vi "HFRR ADV v040.vi"() -> ()   [LabVIEW 2025] (continued)
                }
                n3121 = for {
                  N: 2 -> [_]
                  tunnel: [w3930] -> w3892
                  tunnel: [w3929] -> w3891
                  tunnel: w3886 -> [w3928]
                  tunnel: w3885 -> [w3927]
                  n3122 = call-dynamic "New Report Line.vi"("report in"=w3928, "error in (no error)"=w3927) -> ("report out"=w3930:refnum<class "NI_report.lvclass">, "error out"=w3929:errorcluster)  [unwired: 12 in]
                }
                n3123 = for {
                  N: 25 -> [_]
                  tunnel: w3892 -> [w3926]
                  tunnel: w3891 -> [w3924]
                  tunnel: [w3925] -> w3895
                  tunnel: [w3923] -> w3894
                  n3124 = call-dynamic "Set Report Tab Width.vi"("report in"=w3926, "error in (no error)"=w3924) -> ("report out"=w3925:refnum<class "NI_report.lvclass">, "error out"=w3923:errorcluster)  [unwired: 12 in]
                }
                n3125 = control-ref of="Tab Control 9"() -> (w3890:refnum<vi>)
                n3126 = call-dynamic "Append Control Image to Report.vi"("report in"=w3895, "alignment (default)"=HTML_Report_Image_Alignment."ABSMIDDLE", "ctrl reference"=w3890, "error in (no error)"=w3894) -> ("report out"=w3889:refnum<class "NI_report.lvclass">, "error out"=w3888:errorcluster)  [unwired: 8 in, 2 out]
                n3127 = for {
                  N: 3 -> [_]
                  tunnel: [w3922] -> w3873
                  tunnel: [w3921] -> w3872
                  tunnel: w3889 -> [w3920]
                  tunnel: w3888 -> [w3919]
                  n3128 = call-dynamic "New Report Line.vi"("report in"=w3920, "error in (no error)"=w3919) -> ("report out"=w3922:refnum<class "NI_report.lvclass">, "error out"=w3921:errorcluster)  [unwired: 12 in]
                }
                n3129 = for {
                  N: 100 -> [_]
                  tunnel: w3873 -> [w3918]
                  tunnel: w3872 -> [w3916]
                  tunnel: [w3917] -> w3869
                  tunnel: [w3915] -> w3867
                  n3130 = call-dynamic "Set Report Tab Width.vi"("report in"=w3918, "error in (no error)"=w3916) -> ("report out"=w3917:refnum<class "NI_report.lvclass">, "error out"=w3915:errorcluster)  [unwired: 12 in]
                }
                n3131 = String To Path(string="C:\\LAB-IQ\\im\\Temp_resized.jpg") -> (path=w3859:path)
                n3132 = call-poly <vilib>:"Append Image to Report.vi"("report in"=w3869, "path or URL of image"=w3859, "error in (no error)"=w3867) -> ("report out"=w3868:refnum<class "NI_report.lvclass">, "error out"=w3866:errorcluster)  [unwired: 9 in, 2 out]
                n3133 = call-poly <vilib>:"Open HTML Report in Browser.vi"("report in"=w3868, "error in (no error)"=w3866) -> ("report out"=w3903:refnum<class "NI_report.lvclass">, "error out"=w3902:errorcluster)  [unwired: 11 in, 1 out]
                n3134 = call-dynamic "Dispose Report.vi"("report in"=w3903, "error in (no error)"=w3902) -> ()  [unwired: 13 in, 1 out]
              }
              frame #2 {
              }
              frame #3 {
                n3135 = disable-structure shown="Disabled" {
                  frame Disabled {
                    n3136 = local read "String 10"() -> (w3943:string)
                    n3137 = Concatenate Strings("C:\\LAB-IQ-NXT\\Data\\" ("string"), w3943, ".jpg" ("string")) -> (w3941:string)
                    n3138 = String To Path(string=w3941) -> (path=w3940:path)
                    n3139 = Delete(path (use dialog)=w3940) -> ()  [unwired: 4 in, 3 out]
                  }
                  frame Enabled {
                  }
                }
                n3140 = local write "Print 2"(FALSE ("Print")) -> ()
              }
            }
          }
        }
      }
    }
    n3141 = Wait (ms)(milliseconds to wait=u32 50) -> ()  [unwired: 1 out]
    n3142 = Wait (ms)(milliseconds to wait=u32 50) -> ()  [unwired: 1 out]
    n3143 = local read "Quit"() -> (w2285:bool)
  }
  n3144 = VISA Close(VISA resource name=w43, error in (no error)=w42) -> ()  [unwired: 1 out]
  n3145 = while {
    stop <- w4094 stop-if-true
    n3146 = local read "Auto Start Test"() -> (w4092:bool)
    n3147 = local read "RUN"() -> (w4091:bool)
    n3148 = Wait (ms)(milliseconds to wait=u32 1000) -> ()  [unwired: 1 out]
    n3149 = Or(x=w4091, y=w4092) -> (x .or. y?=w4090:bool)
    n3150 = case shown="True" w4090 {
      frame False {
      }
      frame True {
        n3151 = local read "LVDT STROKE Actual"() -> (w4095:dbl)
        n3152 = In Range and Coerce(upper limit=1.2, x=w4095, lower limit=0.6) -> (In Range?=w4098:bool)  [unwired: 1 out]
        n3153 = call-poly <vilib>:"Random Number (Range).vi"("lower bound (0)"=0.998 ("upper bound (100)"), "upper bound (100)"=1.003) -> ("number"=w4096:dbl)  [unwired: 9 in]
        n3154 = case shown="True" w4098 {
          tunnel: [w4103 w4104] -> w4097
          tunnel: w4096 -> [_ w4104]
          tunnel: w4095 -> [w4103 _]
          frame False {
          }
          frame True {
          }
        }
        "LVDT STROKE DISPLAY" <- w4097
      }
    }
    n3155 = local read "Quit"() -> (w4094:bool)
  }
  n3156 = while {
    tunnel: [w4121] -> w51
    shift-right: [w4114] -> _
    shift-left: 0.0 -> [w4117]
    shift-right: [w4113] -> _
    shift-left: 0.0 -> [w4116]
    shift-right: [w4112] -> _
    shift-left: 100.0 ("vc_cmd") -> [w4115]
    stop <- w4121 stop-if-true
    # "PID LOGIC"
    n3157 = local read "run test Calibration"() -> (w4109:bool)
    n3158 = local read "RUN"() -> (w4119:bool)
    n3159 = local read "Auto Start Temp"() -> (w4110:bool)
    n3160 = local read "Auto Start Test"() -> (w4118:bool)
    n3161 = local read "START TEMP"() -> (w4108:bool)
    n3162 = And(x=w4110, y=w4118) -> (x .and. y?=w4111:bool)
    n3163 = Or(x=w4119, y=w4111) -> (x .or. y?=w4120:bool)
    n3164 = And(x=w4120, y=w4108) -> (x .and. y?=w4107:bool)
    n3165 = And(x=w4109, y=w4108) -> (x .and. y?=w4106:bool)
    n3166 = Or(x=w4106, y=w4107) -> (x .or. y?=w4105:bool)
    n3167 = Wait (ms)(milliseconds to wait="milliseconds to wait") -> ()  [unwired: 1 out]
    n3168 = case shown="True" w4105 {
      tunnel: [400.0 ("out_vc_cmd") w4140] -> w4112
      tunnel: [w4124 w4142] -> w4113
      tunnel: [w4124 w4141] -> w4114
      tunnel: w4117 -> [_ w4131]
      tunnel: w4116 -> [_ w4130]
      tunnel: w4115 -> [_ w4129]
      tunnel: w4109 -> [_ w4125]
      frame False {
        w4124 = 0.0 ("error_out")
      }
      frame True {
        n3169 = case shown="True" w4125 {
          tunnel: [w4149 1.0] -> w4127
          frame False {
            n3170 = local read "Set Strk"() -> (w4148:dbl)
            n3171 = Add(x=w4148, y="Add up Stroke") -> (x+y=w4149:dbl)
          }
          frame True {
          }
        }
        n3172 = local read "LVDT STROKE"() -> (w4126:dbl)
        n3173 = formula code="// Zero-Hardcode Explicit Positional-Form PID Engine\n// Inputs: target_stroke, measured_stroke, dt, prev_error, integral_accumulator_in, prev_vc_cmd\n//         kp, ki, kd, max_step_change, max_amplitude, min_amplitude, startup_cmd\n// Outputs: vc_cmd, error_out, out_error, integral_accumulator_out, out_vc_cmd\n\n// 1. Calculate Tracking Error\nfloat current_error = target_stroke - measured_stroke;\nerror_out = current_error;\n\n// 2. Compute Proportional Term\nfloat p_term = kp * current_error;\n\n// 3. Compute Derivative Term\nfloat d_term = 0.0;\nif (dt > 0.0) {\n    d_term = kd * ((current_error - prev_error) / dt);\n}\n\n// 4. Update and Accumulate Integral Term\nfloat current_integral = integral_accumulator_in + (current_error * dt);\nfloat i_term = ki * current_integral;\n\n// 5. Calculate Ideal Target Command (Anchored by startup baseline)\nfloat ideal_command = startup_cmd + p_term + i_term + d_term;\n\n// 6. Apply Loop Rate Limiting FIRST \n// (Forces the command to climb gradually from prev_vc_cmd instead of jumping straight to max)\nfloat raw_adjustment = ideal_command - prev_vc_cmd;\n\nif (raw_adjustment > max_step_change) {\n    raw_adjustment = max_step_change;\n} else if (raw_adjustment < -max_step_change) {\n    raw_adjustment = -max_step_change;\n}\n\nfloat next_vc_cmd = prev_vc_cmd + raw_adjustment;\n\n// 7. Anti-Windup Protection & Final Output Safety Safeguard Clamping\n// (Back-calculating based on what we are ACTUALLY outputting)\nif (next_vc_cmd > max_amplitude) {\n    float excess = next_vc_cmd - max_amplitude;\n    if (ki > 0.0) {\n        current_integral -= excess / ki;\n    }\n    next_vc_cmd = max_amplitude;\n} else if (next_vc_cmd < min_amplitude) {\n    float excess = next_vc_cmd - min_amplitude;\n    if (ki > 0.0) {\n        current_integral -= excess / ki;\n    }\n    next_vc_cmd = min_amplitude;\n}\n\n// 8. Map to Shift Registers for memory persistence\nvc_cmd = next_vc_cmd;\nout_error = current_error;                   \nintegral_accumulator_out = current_integral;  \nout_vc_cmd = next_vc_cmd;"("target_stroke"=w4127, "measured_stroke"=w4126, "dt"="dt", "integral_accumulator_in"=w4130, "prev_error"=w4131, "prev_vc_cmd"=w4129, "kp"="kp", "ki"="ki", "kd"="kd", "max_step_change"="max_step_change", "max_amplitude"="max_amplitude", "min_amplitude"="min_amplitude", "startup_cmd"="startup_cmd") -> ("vc_cmd"=w4146:dbl, "out_error"=w4141:dbl, "integral_accumulator_out"=w4142:dbl, "out_vc_cmd"=w4140:dbl)  [unwired: 1 out]
        "output Vpp" <- w4146
        n3174 = Number To Fractional String(number=w4146, precision (6)=i16 1) -> (F-format string=w4144:string)  [unwired: 2 in]
        n3175 = Concatenate Strings("DAC;" ("string"), w4144) -> (w4128:string)
        n3176 = local write "Due Write"(w4128) -> ()
        "prev_error" <- w4131
        "integral_accumulator_in" <- w4130
        "prev_vc_cmd" <- w4129
      }
    }
    n3177 = local read "Quit"() -> (w4121:bool)
  }
  n3178 = Or(x=w47, y=w46) -> (x .or. y?=w48:bool)
  n3179 = Or(x=w44, y=w48) -> (x .or. y?=w53:bool)
  n3180 = control-ref of="new picture"() -> ()  [unwired: 1 out]
  n3181 = Or(x=w56, y=w53) -> (x .or. y?=w50:bool)
  n3182 = Or(x=w50, y=w51) -> (x .or. y?=w45:bool)
  n3183 = while {
    tunnel: [w4151] -> w55
    i -> [w4158]
    stop <- w4151 stop-if-true
    n3184 = local read "Quit"() -> (w4151:bool)
    n3185 = Equal To 0?(x=w4158) -> (x = 0?=w4156:bool)
    n3186 = call "Elapsed Time3"("Time Target (s)"=45.0, "Auto Reset"=TRUE) -> ("Time has Elapsed"=w4155:bool)  [unwired: 10 in, 7 out]
    n3187 = Wait (ms)(milliseconds to wait=u32 50) -> ()  [unwired: 1 out]
    n3188 = Or(x=w4155, y=w4156) -> (x .or. y?=w4157:bool)
    n3189 = case shown="True" w4157 {
      frame False {
      }
      frame True {
        n3190 = call <vilib>:"System Exec.vi"("run minimized? (F)"=TRUE, "error in (no error)"="error in (no error)", "command line"="powercfg.exe -change -monitor-timeout-ac 0") -> ("error out"=w4169:errorcluster)  [unwired: 5 in, 3 out]
        n3191 = call <vilib>:"System Exec.vi"("run minimized? (F)"=TRUE, "error in (no error)"=w4169, "command line"="powercfg.exe -change -disk-timeout-ac 0") -> ("error out"=w4168:errorcluster)  [unwired: 5 in, 3 out]
        n3192 = call <vilib>:"System Exec.vi"("run minimized? (F)"=TRUE, "error in (no error)"=w4168, "command line"="powercfg.exe -change -standby-timeout-ac 0") -> ("error out"=w4167:errorcluster)  [unwired: 5 in, 3 out]
        n3193 = call <vilib>:"System Exec.vi"("run minimized? (F)"=TRUE, "error in (no error)"=w4167, "command line"="powercfg.exe -change -hibernate-timeout-ac 0") -> ("error out"=w4166:errorcluster)  [unwired: 5 in, 3 out]
        n3194 = call <vilib>:"Simple Error Handler.vi"("error in (no error)"=w4166) -> ("error out"=w4172:errorcluster)  [unwired: 4 in, 4 out]
        n3195 = call <vilib>:"Clear Errors.vi"("error in (no error)"=w4172) -> ("error out"=→"error out":errorcluster)  [unwired: 5 in, 1 out]
      }
    }
  }
  n3196 = Compound Arithmetic op=OR(w58, w45, w55) -> (w57:bool)
  n3197 = flat-sequence {
    tunnel: w57 -> [_]
    tunnel: [w4174] -> w27
    tunnel: w27 -> [_]
    frame #0 {
      n3198 = call "CLOSE CONNECTION.vi"() -> ("error out"=w4174:errorcluster)  [unwired: 11 in]
    }
    frame #1 {
      n3199 = Quit LabVIEW(quit? (T)=TRUE) -> ()
      n3200 = local write "Quit"(FALSE ("EXIT")) -> ()
    }
  }
  n3201 = property on="Heater Button" class="Bool (strict)"("Visible"=TRUE) -> ()  [unwired: 2 in, 2 out]
  n3202 = while {
    tunnel: [w4181] -> _
    i -> [w4181]
    stop <- w4177 stop-if-true
    # "Langauage selection"
    n3203 = Equal?(x="Lan flag", y=22.0) -> ()  [unwired: 1 out]
    n3204 = disable-structure shown="Disabled" {
      frame Disabled {
        n3205 = stacked-sequence {
          frame #0 {
            n3206 = case shown="\"Russian\"" "Language Selection" {
              tunnel: [0 1] -> w4183
              frame "English", Default {
              }
              frame "Russian" {
              }
            }
            n3207 = for {
              N: 130 -> [_]
              tunnel: "Table" -> [w4192]
              tunnel: w4183 -> [w4191]
              i -> [w4190]
              n3208 = Index Array(array=w4192, index (row)=w4190, index (col)=w4191) -> (element=w4189:string)
              n3209 = case shown="1" w4190 {
                tunnel: w4189 -> [w4193 w4194 _ w4195 w4196 w4197 w4198 w4199 w4200 w4201 w4202 w4203 w4204 w4205 w4206 w4207 w4208 w4209 w4210 w4211 w4212 w4213 w4214 w4215 w4216 w4217 w4218 w4219 w4220 _ _ w4221 w4222 w4223 w4224 w4225 w4226 w4235 w4242 w4249 w4256 w4260 w4263 w4266 w4268 w4270 w4271 w4272 w4273 w4274 w4275 w4276 w4277 w4278 w4279 w4280 w4281 w4282 w4283 w4284 w4285 w4286 w4287 w4288 w4289 w4290 w4291 w4292 w4293 w4294 w4295 w4296 w4297 w4298 w4299 w4300 w4301 w4302 w4303 w4304 w4305 w4306 w4307 w4308 w4309 w4310 w4311 w4312 w4313 w4314 w4315 w4316 w4317 w4318 w4319 w4320 w4321 w4322 w4323 w4324 w4325 w4326 w4327 w4328 w4329 _ w4330 w4331 w4332 w4333 w4334 w4335 w4336 w4337 w4338 w4339 w4340 w4341 w4342 _ w4343 w4344 w4345 w4346 w4347 w4348 _]
                frame 0 {
                  n3210 = local write "S"(w4193) -> ()
                }
                frame 1 {
                  n3211 = local write "S 2"(w4194) -> ()
                }
                frame 2 {
                }
                frame 3 {
                  n3212 = local write "S 4"(w4195) -> ()
                }
                frame 4 {
                  n3213 = property on="FILE" class="Str"("Caption.Text"=w4196) -> ()  [unwired: 2 in, 2 out]
                }
                frame 5 {
                  n3214 = property on="Fuel Discription :" class="Str"("Caption.Text"=w4197) -> ()  [unwired: 2 in, 2 out]
                }
                frame 6 {
                  n3215 = property on="Remarks :" class="Str"("Caption.Text"=w4198) -> ()  [unwired: 2 in, 2 out]
                }
                frame 7 {
                  n3216 = property on="Save & Continue" class="Bool (strict)"("Boolean Text.Text"=w4199) -> ()  [unwired: 2 in, 2 out]
                }
                frame 8 {
                }
                frame 9 {
                  n3217 = property on="Set Hz" class="DigNum (strict)"("Caption.Text"=w4201) -> ()  [unwired: 2 in, 2 out]
                }
                frame 10 {
                }
                frame 11 {
                  n3218 = property on="NORMAL LOAD" class="DigNum (strict)"("Caption.Text"=w4203) -> ()  [unwired: 2 in, 2 out]
                }
                frame 12 {
                }
                frame 13 {
                  n3219 = property on="Set Temp" class="DigNum (strict)"("Caption.Text"=w4205) -> ()  [unwired: 2 in, 2 out]
                }
                frame 14 {
                  n3220 = local write "S 15"(w4206) -> ()
                }
                frame 15 {
                  n3221 = property on="Set Rh" class="DigNum (strict)"("Caption.Text"=w4207) -> ()  [unwired: 2 in, 2 out]
                }
                frame 16 {
                }
                frame 17 {
                  n3222 = local write "S 18"(w4209) -> ()
                }
                frame 18 {
                  "String 17" <- w4210
                }
                frame 19 {
                  n3223 = property on="test time" class="DigNum (strict)"("Caption.Text"=w4211) -> ()  [unwired: 2 in, 2 out]
                }
                frame 20 {
                  "String 18" <- w4212
                  "String 22" <- w4212
                }
                frame 21 {
                  n3224 = property on="Elapsed time" class="DigNum (strict)"("Caption.Text"=w4213) -> ()  [unwired: 2 in, 2 out]
                }
                frame 22 {
                  n3225 = property on="Samplingtime 2" class="DigNum (strict)"("Caption.Text"=w4214) -> ()  [unwired: 2 in, 2 out]
                }
                frame 23 {
                  "String 21" <- w4215
                }
                frame 24 {
                  n3226 = property on="Countdown" class="DigNum (strict)"("Caption.Text"=w4216) -> ()  [unwired: 2 in, 2 out]
                }
                frame 25 {
                  n3227 = property on="Countdown 2" class="DigNum (strict)"("Caption.Text"=w4217) -> ()  [unwired: 2 in, 2 out]
                }
                frame 26 {
                  n3228 = property on="Engage" class="Bool (strict)"("Boolean Text.Text"=w4218) -> ()  [unwired: 2 in, 2 out]
                }
                frame 27 {
                  n3229 = property on="Boolean  4" class="Bool (strict)"("Boolean Text.Text"=w4219) -> ()  [unwired: 2 in, 2 out]
                }
                frame 28 {
                  n3230 = property on="Test \nStatus" class="Bool (strict)"("Boolean Text.Text"=w4220) -> ()  [unwired: 2 in, 2 out]
                }
                frame 29 {
                }
                frame 30 {
                }
                frame 31 {
                }
                frame 32 {
                  n3231 = property on="RSTCOF" class="Bool"("Boolean Text.Text"=w4222) -> ()  [unwired: 2 in, 2 out]
                  n3232 = property on="RST FF" class="Bool"("Boolean Text.Text"=w4222) -> ()  [unwired: 2 in, 2 out]
                  n3233 = property on="RST TEMP" class="Bool"("Boolean Text.Text"=w4222) -> ()  [unwired: 2 in, 2 out]
                  n3234 = property on="RSTV1 3" class="Bool"("Boolean Text.Text"=w4222) -> ()  [unwired: 2 in, 2 out]
                  n3235 = property on="rstv2" class="Bool"("Boolean Text.Text"=w4222) -> ()  [unwired: 2 in, 2 out]
                  n3236 = property on="RSTV1 2" class="Bool"("Boolean Text.Text"=w4222) -> ()  [unwired: 2 in, 2 out]
                  n3237 = property on="RST CP" class="Bool"("Boolean Text.Text"=w4222) -> ()  [unwired: 2 in, 2 out]
                }
                frame 33 {
                  "S 61" <- w4223
                }
                frame 34 {
                  "String 23" <- w4224
                }
                frame 35 {
                  n3238 = property on="Rh Before" class="DigNum (strict)"("Caption.Text"=w4225) -> ()  [unwired: 2 in, 2 out]
                }
                frame 36 {
                  n3239 = Match Pattern(string=w4226, regular expression=",") -> (before substring=→"bs":string, after substring=→"as":string)  [unwired: 1 in, 2 out]
                  n3240 = property on="Rh After" class="DigNum (strict)"("Caption.Text"=w4226) -> ()  [unwired: 2 in, 2 out]
                }
                frame 37 {
                  n3241 = Match Pattern(string=w4235, regular expression=",") -> (before substring=w4234:string, after substring=w4233:string)  [unwired: 1 in, 2 out]
                  "bs" <- w4234
                  "as" <- w4233
                  n3242 = Concatenate Strings(w4234, w4233) -> (w4230:string)
                  n3243 = property on="Humidity before test 2" class="DigNum (strict)"("Caption.Text"=w4230) -> ()  [unwired: 2 in, 2 out]
                  n3244 = Concatenate Strings(w4230, "=" ("string")) -> (w4231:string)
                  n3245 = local write "S 38"(w4231) -> ()
                }
                frame 38 {
                  n3246 = Match Pattern(string=w4242, regular expression=",") -> (before substring=w4241:string, after substring=w4240:string)  [unwired: 1 in, 2 out]
                  "bs" <- w4241
                  "as" <- w4240
                  n3247 = Concatenate Strings(w4241, w4240) -> (w4237:string)
                  n3248 = property on="Humidity after test 2" class="DigNum (strict)"("Caption.Text"=w4237) -> ()  [unwired: 2 in, 2 out]
                  n3249 = Concatenate Strings(w4237, "=" ("string")) -> (w4239:string)
                  n3250 = local write "S 39"(w4239) -> ()
                }
                frame 39 {
                  n3251 = Match Pattern(string=w4249, regular expression=",") -> (before substring=w4248:string, after substring=w4247:string)  [unwired: 1 in, 2 out]
                  "bs" <- w4248
                  "as" <- w4247
                  n3252 = Concatenate Strings(w4248, w4247) -> (w4244:string)
                  n3253 = property on="Temperature before test 2" class="DigNum (strict)"("Caption.Text"=w4244) -> ()  [unwired: 2 in, 2 out]
                  n3254 = Concatenate Strings(w4244, "=" ("string")) -> (→"String 34":string)
                }
                frame 40 {
                  n3255 = Match Pattern(string=w4256, regular expression=",") -> (before substring=w4255:string, after substring=w4254:string)  [unwired: 1 in, 2 out]
                  "bs" <- w4255
                  "as" <- w4254
                  n3256 = Concatenate Strings(w4255, w4254) -> (w4251:string)
                  n3257 = property on="Temperature after test 2" class="DigNum (strict)"("Caption.Text"=w4251) -> ()  [unwired: 2 in, 2 out]
                  n3258 = Concatenate Strings(w4251, "=" ("string")) -> (→"String 35":string)
                  n3259 = property on="Temperature after test" class="DigNum (strict)"("Caption.Text"=w4251) -> ()  [unwired: 2 in, 2 out]
                }
                frame 41 {
                  n3260 = property on="AVP 2" class="DigNum (strict)"("Caption.Text"=w4260) -> ()  [unwired: 2 in, 2 out]
                  n3261 = Concatenate Strings(w4260, "=" ("string")) -> (→"String 36":string)
                }
                frame 42 {
                  n3262 = property on="MWSD 2" class="DigNum (strict)"("Caption.Text"=w4263) -> ()  [unwired: 2 in, 2 out]
                  n3263 = Concatenate Strings(w4263, "=" ("string")) -> (→"String 37":string)
                }
                frame 43 {
                  n3264 = property on="HCF 2" class="DigNum (strict)"("Caption.Text"=w4266) -> ()  [unwired: 2 in, 2 out]
                  n3265 = Concatenate Strings(w4266, "=" ("string")) -> (→"String 38":string)
                }
                frame 44 {
                  n3266 = Concatenate Strings(w4268, "=" ("string")) -> (→"String 39":string)
                  n3267 = property on="WS1.4 2" class="DigNum (strict)"("Caption.Text"=w4268) -> ()  [unwired: 2 in, 2 out]
                }
                frame 45 {
                }
                frame 46 {
                  n3268 = local write "S 47"(w4271) -> ()
                }
                frame 47 {
                  n3269 = local write "S 48"(w4272) -> ()
                }
                frame 48 {
                  n3270 = local write "S 49"(w4273) -> ()
                }
                frame 49 {
                  n3271 = local write "S 50"(w4274) -> ()
                }
                frame 50 {
                  n3272 = local write "S 51"(w4275) -> ()
                }
                frame 51 {
                  n3273 = local write "S 52"(w4276) -> ()
                }
                frame 52 {
                  n3274 = local write "S 53"(w4277) -> ()
                }
                frame 53 {
                  n3275 = local write "S 54"(w4278) -> ()
                }
                frame 54 {
                  n3276 = local write "S 55"(w4279) -> ()
                }
                frame 55 {
                  n3277 = local write "S 56"(w4280) -> ()
                }
                frame 56 {
                  n3278 = local write "S 57"(w4281) -> ()
                }
                frame 57 {
                  n3279 = local write "S 58"(w4282) -> ()
                }
                frame 58 {
                  n3280 = local write "S 59"(w4283) -> ()
                }
                frame 59 {
                  n3281 = local write "S 60"(w4284) -> ()
                }
                frame 60 {
                  n3282 = local write "S 62"(w4285) -> ()
                }
                frame 61 {
                  n3283 = local write "S 63"(w4286) -> ()
                }
                frame 62 {
                  n3284 = local write "S 64"(w4287) -> ()
                }
                frame 63 {
                  n3285 = local write "S 65"(w4288) -> ()
                }
                frame 64 {
                  n3286 = local write "S 66"(w4289) -> ()
                }
                frame 65 {
                  n3287 = local write "S 67"(w4290) -> ()
                }
                frame 66 {
                  n3288 = local write "S 68"(w4291) -> ()
                }
                frame 67 {
                  n3289 = local write "S 69"(w4292) -> ()
                }
                frame 68 {
                  n3290 = local write "S 70"(w4293) -> ()
                }
                frame 69 {
                  n3291 = local write "S 71"(w4294) -> ()
                }
                frame 70 {
                  n3292 = local write "S 72"(w4295) -> ()
                }
                frame 71 {
                  n3293 = local write "S 73"(w4296) -> ()
                }
                frame 72 {
                  n3294 = local write "S 74"(w4297) -> ()
                }
                frame 73 {
                  n3295 = local write "S 75"(w4298) -> ()
                }
                frame 74 {
                  n3296 = local write "S 76"(w4299) -> ()
                }
                frame 75 {
                  n3297 = local write "S 77"(w4300) -> ()
                }
                frame 76 {
                  n3298 = local write "S 78"(w4301) -> ()
                }
                frame 77 {
                  n3299 = local write "S 79"(w4302) -> ()
                }
                frame 79 {
                  n3300 = property on="Sample Temperature ( °C )" class="XYGraph (strict)"("Y Scale.Name Label.Text"=w4303) -> ()  [unwired: 2 in, 2 out]
                }
                frame 80 {
                  n3301 = local write "S 81"(w4304) -> ()
                  n3302 = property on="Humidity ( %RH )" class="XYGraph (strict)"("Y Scale.Name Label.Text"=w4304) -> ()  [unwired: 2 in, 2 out]
                }
                frame 78 {
                  n3303 = property on="Air Temperature  ( °C )" class="XYGraph (strict)"("X Scale.Name Label.Text"=w4305) -> ()  [unwired: 2 in, 2 out]
                  n3304 = property on="Humidity ( %RH )" class="XYGraph (strict)"("X Scale.Name Label.Text"=w4305) -> ()  [unwired: 2 in, 2 out]
                  n3305 = property on="Sample Temperature ( °C )" class="XYGraph (strict)"("X Scale.Name Label.Text"=w4305) -> ()  [unwired: 2 in, 2 out]
                  n3306 = property on="Coefficient Of Friction" class="XYGraph (strict)"("X Scale.Name Label.Text"=w4305) -> ()  [unwired: 2 in, 2 out]
                }
                frame 81 {
                  n3307 = property on="Air Temperature  ( °C )" class="XYGraph (strict)"("Y Scale.Name Label.Text"=w4306) -> ()  [unwired: 2 in, 2 out]
                }
                frame 82 {
                  n3308 = local write "S 84"(w4307) -> ()
                }
                frame 83 {
                  n3309 = local write "S 85"(w4308) -> ()
                }
                frame 84 {
                  n3310 = local write "S 86"(w4309) -> ()
                }
                frame 85 {
                  n3311 = local write "S 87"(w4310) -> ()
                }
                frame 86 {
                  n3312 = local write "S 88"(w4311) -> ()
                }
                frame 87 {
                }
                frame 88 {
                  n3313 = local write "S 90"(w4313) -> ()
                }
                frame 89 {
                  n3314 = local write "S 91"(w4314) -> ()
                }
                frame 90 {
                  n3315 = local write "S 92"(w4315) -> ()
                }
                frame 91 {
                  n3316 = local write "S 93"(w4316) -> ()
                }
                frame 92 {
                  n3317 = local write "S 94"(w4317) -> ()
                }
                frame 93 {
                  n3318 = local write "S 95"(w4318) -> ()
                }
                frame 94 {
                  n3319 = local write "S 96"(w4319) -> ()
                }
                frame 95 {
                  n3320 = local write "S 97"(w4320) -> ()
                }
                frame 96 {
                  n3321 = local write "S 98"(w4321) -> ()
                }
                frame 97 {
                  n3322 = local write "S 99"(w4322) -> ()
                }
                frame 98 {
                  n3323 = local write "S 100"(w4323) -> ()
                }
                frame 99 {
                  n3324 = local write "S 101"(w4324) -> ()
                }
                frame 100 {
                  n3325 = local write "S 102"(w4325) -> ()
                }
                frame 101 {
                  n3326 = local write "S 103"(w4326) -> ()
                }
                frame 102 {
                  n3327 = local write "S 104"(w4327) -> ()
                }
                frame 103 {
                  n3328 = local write "S 105"(w4328) -> ()
                }
                frame 104 {
                  n3329 = local write "S 106"(w4329) -> ()
                }
                frame 105 {
                }
                frame 106 {
                  n3330 = property on="OK Button 17" class="Bool (strict)"("Boolean Text.Text"=w4330) -> ()  [unwired: 2 in, 2 out]
                }
                frame 107 {
                  n3331 = property on="OK Button 16" class="Bool (strict)"("Boolean Text.Text"=w4331) -> ()  [unwired: 2 in, 2 out]
                }
                frame 108 {
                  n3332 = property on="TITTLE" class="Str"("Caption.Text"=w4332) -> ()  [unwired: 2 in, 2 out]
                }
                frame 109 {
                  "String 30" <- w4333
                }
                frame 110 {
                  n3333 = property on="Test Date" class="Str"("Caption.Text"=w4334) -> ()  [unwired: 2 in, 2 out]
                  "String 31" <- w4334
                }
                frame 111 {
                  n3334 = property on="Sample ID" class="Str"("Caption.Text"=w4335) -> ()  [unwired: 2 in, 2 out]
                  "String 32" <- w4335
                }
                frame 112 {
                  n3335 = property on="Tested by" class="Str"("Caption.Text"=w4336) -> ()  [unwired: 2 in, 2 out]
                  "String 33" <- w4336
                }
                frame 113 {
                  n3336 = property on="System Configured Printers 2" class="Arr (strict)"("Caption.Text"=w4337) -> ()  [unwired: 2 in, 2 out]
                }
                frame 114 {
                  n3337 = property on="Selected Printer" class="Str"("Caption.Text"=w4338) -> ()  [unwired: 2 in, 2 out]
                }
                frame 115 {
                  n3338 = property on="Select Printer 3" class="DigNum (strict)"("Caption.Text"=w4339) -> ()  [unwired: 2 in, 2 out]
                }
                frame 116 {
                  n3339 = property on="Print" class="Bool (strict)"("Boolean Text.Text"=w4340) -> ()  [unwired: 2 in, 2 out]
                }
                frame 117 {
                  "String 41" <- w4341
                }
                frame 118 {
                  n3340 = property on="tested by" class="Str"("Caption.Text"=w4342) -> ()  [unwired: 2 in, 2 out]
                }
                frame 119 {
                }
                frame 120 {
                  n3341 = property on="Export" class="Bool (strict)"("Boolean Text.Text"=w4343) -> ()  [unwired: 2 in, 2 out]
                }
                frame 121 {
                }
                frame 122 {
                }
                frame 123 {
                  n3342 = property on="Select File Type" class="Enum (strict)"("Caption.Text"=w4346) -> ()  [unwired: 2 in, 2 out]
                }
                frame 124 {
                  n3343 = property on="s.NO" class="Str"("Caption.Text"=w4347) -> ()  [unwired: 2 in, 2 out]
                  "String 45" <- w4347
                }
                frame 125 {
                  n3344 = property on="trip1 8" class="Bool (strict)"("Boolean Text.Text"=w4348) -> ()  [unwired: 2 in, 2 out]
                }
                frame 126, Default {
                }
              }
            }
          }
          frame #1 {
            w4356 = TRUE ("Visible")
            n3345 = local read "S 91"() -> (w4373:string)
            n3346 = local read "S 90"() -> (w4372:string)
            n3347 = local read "S 88"() -> (w4371:string)
            n3348 = property on="File Path" class="Path"("Caption.Text"=w4372) -> ()  [unwired: 2 in, 2 out]
            n3349 = local read "S 71"() -> (w4366:string)
            n3350 = local read "S 86"() -> (w4368:string)
            n3351 = local read "S 85"() -> (w4369:string)
            n3352 = local read "S 87"() -> (w4367:string)
            n3353 = local read "S 84"() -> (w4370:string)
            n3354 = local read "S 103"() -> (w4355:string)
            n3355 = local read "S 104"() -> (w4354:string)
            n3356 = property on="Password" class="Str"("Caption.Text"=w4369) -> ()  [unwired: 2 in, 2 out]
            n3357 = property on="EDIT" class="Bool (strict)"("Boolean Text.Text"=w4366) -> ()  [unwired: 2 in, 2 out]
            n3358 = property on="SAVE" class="Bool (strict)"("Boolean Text.Text"=w4370) -> ()  [unwired: 2 in, 2 out]
            n3359 = Build Array(w4355, w4354) -> (w4353:string[])
            n3360 = property on="Heater Button" class="Bool (strict)"("Strings [4]"=w4353) -> ()  [unwired: 2 in, 2 out]
            n3361 = local read "S 92"() -> (w4365:string)
            n3362 = local read "S 93"() -> (w4364:string)
            n3363 = local read "S 105"() -> (w4351:string)
            n3364 = local read "S 106"() -> (w4350:string)
            n3365 = Build Array(w4365, w4364) -> ()  [unwired: 1 out]
            n3366 = Build Array(w4351, w4350) -> (w4352:string[])
            n3367 = local read "S 95"() -> (w4362:string)
            n3368 = local read "S 94"() -> (w4363:string)
            n3369 = local read "bs"() -> (w4378:string)
            n3370 = local read "as"() -> (w4379:string)
            n3371 = property on="Humidity" class="Bool (strict)"("Strings [4]"=w4352) -> ()  [unwired: 2 in, 2 out]
            n3372 = Concatenate Strings(w4378, "\r", w4379) -> ()  [unwired: 1 out]
            n3373 = property on="Rh After" class="DigNum (strict)"("Caption.Size to Text?"=TRUE ("Caption.Size to Text")) -> ()  [unwired: 2 in, 2 out]
            n3374 = local read "S 48"() -> (w4402:string)
            n3375 = local read "S 50"() -> (w4400:string)
            n3376 = local read "S 51"() -> (w4399:string)
            n3377 = local read "S 49"() -> (w4401:string)
            n3378 = local read "S 52"() -> (w4398:string)
            n3379 = local read "as"() -> (w4383:string)
            n3380 = local read "bs"() -> (w4384:string)
            n3381 = local read "S 56"() -> (w4397:string)
            n3382 = local read "S 57"() -> (w4396:string)
            n3383 = local read "S 58"() -> (w4395:string)
            n3384 = local read "S 59"() -> (w4394:string)
            n3385 = property on="OPEN" class="Bool (strict)"("Boolean Text.Text"=w4398) -> ()  [unwired: 2 in, 2 out]
            n3386 = property on="OPEN 1" class="Bool (strict)"("Boolean Text.Text"=w4402) -> ()  [unwired: 2 in, 2 out]
            n3387 = property on="OPEN 2" class="Bool (strict)"("Boolean Text.Text"=w4401) -> ()  [unwired: 2 in, 2 out]
            n3388 = property on="OPEN 3" class="Bool (strict)"("Boolean Text.Text"=w4400) -> ()  [unwired: 2 in, 2 out]
            n3389 = property on="OPEN 4" class="Bool (strict)"("Boolean Text.Text"=w4399) -> ()  [unwired: 2 in, 2 out]
            n3390 = Concatenate Strings(w4384, "\r", w4383) -> ()  [unwired: 1 out]
            n3391 = local read "S 102"() -> (w4357:string)
            n3392 = property on="КОФ1" class="DigNum (strict)"("Caption.Text"=w4397) -> ()  [unwired: 2 in, 2 out]
            n3393 = local read "S 98"() -> (w4361:string)
            n3394 = local read "S 99"() -> (w4360:string)
            n3395 = local read "S 100"() -> (w4359:string)
            n3396 = local read "S 101"() -> (w4358:string)
            n3397 = property on="КОФ2" class="DigNum (strict)"("Caption.Text"=w4396) -> ()  [unwired: 2 in, 2 out]
            n3398 = property on="КОФ3" class="DigNum (strict)"("Caption.Text"=w4395) -> ()  [unwired: 2 in, 2 out]
            n3399 = property on="КОФ4" class="DigNum (strict)"("Caption.Text"=w4394) -> ()  [unwired: 2 in, 2 out]
            n3400 = local read "bs"() -> (w4382:string)
            n3401 = local read "as"() -> (w4381:string)
            n3402 = local read "S 60"() -> (w4393:string)
            n3403 = local read "S 54"() -> (w4403:string)
            n3404 = Concatenate Strings(w4382, "\r", w4381) -> ()  [unwired: 1 out]
            n3405 = Concatenate Strings(w4403, w4393) -> ()  [unwired: 1 out]
            n3406 = local read "S 77"() -> (→"String 43":string)
            n3407 = local read "S 76"() -> (w4376:string)
            n3408 = local read "S 78"() -> (w4375:string)
            n3409 = local read "S 71"() -> (w4387:string)
            n3410 = local read "S 66"() -> (w4392:string)
            n3411 = local read "S 67"() -> (w4391:string)
            n3412 = local read "S 68"() -> (w4390:string)
            n3413 = local read "S 69"() -> (w4389:string)
            n3414 = local read "S 70"() -> (w4388:string)
            n3415 = property on="AIR TEMP" class="DigNum (strict)"("Caption.Text"=w4375) -> ()  [unwired: 2 in, 2 out]
            n3416 = property on="Set Strk" class="DigNum (strict)"("Caption.Text"=w4376) -> ()  [unwired: 2 in, 2 out]
            n3417 = property on="SPEED OUT:" class="DigNum (strict)"("Caption.Text"=w4390) -> ()  [unwired: 2 in, 2 out]
            n3418 = property on="EDIT" class="Bool (strict)"("Boolean Text.Text"=w4387) -> ()  [unwired: 2 in, 2 out]
            n3419 = local read "S 79"() -> (w4374:string)
          }
          frame #2 {
          }
        }
        n3420 = local write "Lan flag"(10.0 ("Lan flag")) -> ()
      }
      frame Enabled {
      }
    }
    n3421 = Wait (ms)(milliseconds to wait=u32 2000) -> ()  [unwired: 1 out]
    n3422 = local read "Quit"() -> (w4177:bool)
  }
  n3423 = while {
    shift-right: [w4409] -> _
    shift-left: _ -> [w4410]
    shift-right: [w4407] -> _
    shift-left: T18 {"Read Heave and Surge"="", "Bytes at Heave Port"=0.0, "Heave and Surge COM Port:"="COM9", "Com Port 2"="COM7", "Residual Due"="", "Heave COM Status 2"=TRUE, "Heave COM Status"=TRUE, "Port 2"=TRUE, "Sway PPR"=6400.0, "Surge PPR"=6400.0, "Heave PPR"=6400.0, "Sway Pitch"=2.0, "Surge Pitch"=3.0, "Heave Pitch"=4.0, "Sway Pulses/mm"=320.0, "Surge Pulses/mm"=1600.0, "Heave Pulses/mm"=1600.0, "inner loop"=0.0, "Read Heave and Surge 2"="", "String 36"="", "Write S"=FALSE, "WriteCC1"=[""], "Heave COM Loop"=0, "LastCom"="", "EXIT"=FALSE, "Error Heave"={"status"=TRUE, "code"=-1073807343, "source"=""}} -> [w4406]
    shift-right: [w4404] -> _
    shift-left: enum16{"init", "MAIN", "Panel Close"}."init" -> [w4405]
    stop <- w4408 stop-if-true
    # "HUMIDITY LOOP LOGIC"
    n3424 = case shown="\"MAIN\"" w4405 {
      tunnel: w4410 -> [w4424 w4448 w4512 w4514]
      tunnel: [w4419 w4435 w4512 w4514] -> w4409
      tunnel: [_ _ TRUE _] -> w4408
      tunnel: [w4416 w4433 w4510 w4513] -> w4407
      tunnel: w4406 -> [w4421 w4447 w4510 w4513]
      tunnel: [enum16{"init", "MAIN", "Panel Close"}."MAIN" w4442 _ _] -> w4404
      frame "init" {
        n3425 = local read "C3 :"() -> (w4411:refnum<visa-resource-name>)
        n3426 = Bundle By Name(cluster=w4421, "Heave and Surge COM Port:"=w4411) -> (w4420:T18)
        n3427 = call "Instrument fgv uno.vi"("Enum"=T32."INIT", "error in (no error) 2"=w4424, "INPUT"=w4420) -> ("error"=w4422:errorcluster, "output"=w4418:T18)  [unwired: 6 in, 1 out]
        n3428 = case shown="Error" w4422 {
          selector: w4422 -> [w4426 _]
          tunnel: [w4426 w4430] -> w4419
          tunnel: w4418 -> [w4425 w4428]
          tunnel: [w4425 w4427] -> w4417
          frame No Error {
          }
          frame Error {
            n3429 = call "Instrument fgv uno.vi"("Enum"=T32."ERROR INIT", "INPUT"=w4428) -> ("error"=w4431:errorcluster, "output"=w4427:T18)  [unwired: 7 in, 1 out]
            n3430 = call <vilib>:"Clear Errors.vi"("error in (no error)"=w4431) -> ("error out"=w4430:errorcluster)  [unwired: 5 in, 1 out]
          }
        }
        n3431 = local read "LastCom Humidity"() -> (w4414:string)
        n3432 = Unbundle By Name(w4417) -> ("Heave COM Status 2"=→"COM Status":bool, "Error Heave"=→"Error":errorcluster)  [unwired: 1 out]
        n3433 = Bundle By Name(cluster=w4417, "LastCom"=w4414) -> (w4416:T18)
      }
      frame "MAIN" {
        n3434 = Unbundle By Name(w4447) -> ("Com Port 2"=w4437:refnum<visa-resource-name>)
        n3435 = local read "C3 :"() -> (w4438:refnum<visa-resource-name>)
        n3436 = local write "COM Port Humidity :"(w4437) -> ()
        n3437 = Bundle By Name(cluster=w4447, "Heave and Surge COM Port:"=w4438) -> (w4446:T18)
        n3438 = Equal?(x=w4437, y=w4438) -> (x = y?=w4451:bool)
        n3439 = case shown="True" w4451 {
          tunnel: [w4466 w4483] -> w4436
          tunnel: w4448 -> [w4467 w4489]
          tunnel: w4446 -> [w4465 w4487]
          tunnel: [w4464 w4482] -> w4434
          frame False {
            n3440 = call <vilib>:"Clear Errors.vi"("error in (no error)"=w4467) -> ("error out"=w4463:errorcluster)  [unwired: 5 in, 1 out]
            n3441 = call "Instrument fgv uno.vi"("Enum"=T32."ERROR INIT", "error in (no error) 2"=w4463, "INPUT"=w4465) -> ("error"=w4469:errorcluster, "output"=w4464:T18)  [unwired: 6 in, 1 out]
            n3442 = call <vilib>:"Clear Errors.vi"("error in (no error)"=w4469) -> ("error out"=w4466:errorcluster)  [unwired: 5 in, 1 out]
          }
          frame True {
            n3443 = call "Instrument fgv uno.vi"("Enum"=T32."READ", "error in (no error) 2"=w4489, "INPUT"=w4487) -> ("error"=w4488:errorcluster, "output"=w4481:T18)  [unwired: 6 in, 1 out]
            n3444 = Bundle By Name(cluster=w4481, "String 36"="WRITE HUMIDITY") -> (w4480:T18)
            n3445 = case shown="True" "Write Humidity" {
              selector: "Write Humidity" -> [_ w4509]
              tunnel: w4488 -> [w4502 w4508]
              tunnel: [w4502 w4507] -> w4478
              tunnel: w4480 -> [w4501 w4505]
              tunnel: [w4501 w4504] -> w4477
              frame False {
              }
              frame True {
                n3446 = Not(x=w4509) -> (.not. x?=w4503:bool)
                n3447 = local write "Write Humidity"(w4503) -> ()
                n3448 = call "Instrument fgv uno.vi"("Enum"=T32."MANUAL WRITE", "error in (no error) 2"=w4508, "INPUT"=w4505) -> ("error"=w4507:errorcluster, "output"=w4504:T18)  [unwired: 6 in, 1 out]
              }
            }
            n3449 = Array Size(array="WriteHumidity") -> (size(s)=w4475:i32)
            n3450 = Greater Than 0?(x=w4475) -> (x > 0?=w4474:bool)
            n3451 = call "Instrument fgv uno.vi"("Enum"=T32."WRITE", "error in (no error) 2"=w4478, "WriteCC1"="WriteHumidity", "INPUT"=w4477) -> ("error"=w4485:errorcluster, "WriteCC1 2"=w4476:string[], "output"=w4484:T18)  [unwired: 5 in]
            n3452 = case shown="True" w4474 {
              tunnel: w4476 -> [_ w4491]
              frame False {
              }
              frame True {
                n3453 = local write "WriteHumidity"(w4491) -> ()
              }
            }
            n3454 = case shown="No Error" w4485 {
              selector: w4485 -> [w4492 w4495]
              tunnel: w4484 -> [w4493 w4500]
              tunnel: [w4493 w4499] -> w4482
              tunnel: [w4492 w4497] -> w4483
              frame No Error {
              }
              frame Error {
                n3455 = call <vilib>:"Clear Errors.vi"("error in (no error)"=w4495) -> ("error out"=w4494:errorcluster)  [unwired: 5 in, 1 out]
                n3456 = call "Instrument fgv uno.vi"("Enum"=T32."ERROR INIT", "error in (no error) 2"=w4494, "INPUT"=w4500) -> ("error"=w4498:errorcluster, "output"=w4499:T18)  [unwired: 6 in, 1 out]
                n3457 = call <vilib>:"Clear Errors.vi"("error in (no error)"=w4498) -> ("error out"=w4497:errorcluster)  [unwired: 5 in, 1 out]
              }
            }
            n3458 = Unbundle By Name(w4482) -> ("LastCom"=→"LastCom Humidity":string, "Read Heave and Surge"=→"Read HUMIDITY":string)
          }
        }
        n3459 = Unbundle By Name(w4434) -> ("Heave COM Status 2"=w4450:bool, "Error Heave"=w4439:errorcluster, "Bytes at Heave Port"=→"Bytes at Humidity Port  2":dbl)  [unwired: 1 out]
        n3460 = Unbundle By Name(w4439) -> ("status"=→"Humidity Port":bool)
        n3461 = Not(x=w4450) -> (.not. x?=w4440:bool)
        n3462 = local write "Error"(w4439) -> ()
        n3463 = local read "Quit"() -> (w4443:bool)
        n3464 = local write "COM Status"(w4440) -> ()
        n3465 = Select(t=enum16{"init", "MAIN", "Panel Close"}."Panel Close", s=w4443, f=enum16{"init", "MAIN", "Panel Close"}."MAIN") -> (s? t:f=w4442:enum16{"init", "MAIN", "Panel Close"})
        n3466 = local read "Humidity 2"() -> (w4432:bool)
        n3467 = case shown="True" w4432 {
          selector: w4432 -> [_ w4454]
          tunnel: w4436 -> [w4452 w4459]
          tunnel: [w4452 w4458] -> w4435
          tunnel: w4434 -> [w4453 w4457]
          tunnel: [w4453 w4456] -> w4433
          frame False {
          }
          frame True {
            n3468 = Not(x=w4454) -> (.not. x?=→"Humidity 2":bool)
            n3469 = call <vilib>:"Clear Errors.vi"("error in (no error)"=w4459) -> ("error out"=w4462:errorcluster)  [unwired: 5 in, 1 out]
            n3470 = call "Instrument fgv uno.vi"("Enum"=T32."ERROR INIT", "error in (no error) 2"=w4462, "INPUT"=w4457) -> ("error"=w4460:errorcluster, "output"=w4456:T18)  [unwired: 6 in, 1 out]
            n3471 = call <vilib>:"Clear Errors.vi"("error in (no error)"=w4460) -> ("error out"=w4458:errorcluster)  [unwired: 5 in, 1 out]
          }
        }
      }
      frame "Panel Close" {
      }
      frame Default {
      }
    }
  }
  n3472 = while {
    stop <- w4516 stop-if-true
    n3473 = call <vilib>:"High Resolution Polling Wait.vi"("seconds to wait"=0.05) -> ()  [unwired: 10 in, 1 out]
    n3474 = disable-structure shown="Enabled" {
      frame Disabled {
        n3475 = local read "Read HUMIDITY"() -> (w4517:string)
        n3476 = Spreadsheet String To Array(delimiter (Tab)=",", format string="", spreadsheet string=w4517, array type (2D Dbl)=string[] []) -> (array=w4536:string[])
        n3477 = for {
          tunnel: w4536 -> [w4545] mode=indexing
          tunnel: string[] ["STATE;", "SET;", "RH;", "T;", "AMB_RH;", "AMB_T;", "PUMP;", "FAN_IN;", "FAN_OUT;", "DEHUM;", "CURRENT;", "STALL;"] -> [w4544] mode=indexing
          tunnel: [w4543] -> w4535 mode=indexing
          n3478 = Match Pattern(string=w4545, regular expression=w4544) -> (after substring=w4543:string)  [unwired: 1 in, 3 out]
        }
        n3479 = Index Array(array=w4535) -> (element #1=w4534:string, element #2=w4533:string, element #3=w4525:string, element #4=w4524:string, element #5=w4523:string, element #6=w4532:string, element #7=w4531:string, element #8=w4530:string, element #9=w4529:string, element #10=w4528:string, element #11=w4527:string, element #12=w4526:string)  [unwired: 12 in]
        n3480 = Fract/Exp String To Number(string=w4525) -> (number=w4518:dbl)  [unwired: 3 in, 1 out]
        n3481 = Fract/Exp String To Number(string=w4523) -> (number=w4522:dbl)  [unwired: 3 in, 1 out]
        n3482 = local write "Ambient Humidity :"(w4522) -> ()
        n3483 = Equal?(x=w4518, y=0.0) -> (x = y?=w4520:bool)
        n3484 = case shown="True" w4520 {
          tunnel: [w4541 w4542] -> w4519
          tunnel: w4518 -> [w4541 _]
          frame False {
            (unwired) 0.0
            "Humidity temp" <- w4541
          }
          frame True {
            n3485 = local read "Humidity temp"() -> (w4542:dbl)
          }
        }
        "RH Numeric:" <- w4519
      }
      frame Enabled {
        n3486 = local read "Read HUMIDITY"() -> (w4565:string)
        n3487 = Spreadsheet String To Array(delimiter (Tab)=",", format string="", spreadsheet string=w4565, array type (2D Dbl)=dbl[] []) -> (array=w4561:dbl[])
        n3488 = Index Array(array=w4561) -> (element #1=→"STATE :":dbl, element #2=→"SET :":dbl, element #3=w4546:dbl, element #4=→"T :":dbl, element #5=→"AMB_RH :":dbl, element #6=→"AMB_T :":dbl, element #7=→"PUMP :":dbl, element #8=→"FAN_IN :":dbl, element #9=→"FAN_OUT :":dbl, element #10=→"DEHUM :":dbl, element #11=→"CURRENT :":dbl, element #12=→"STALL":dbl)  [unwired: 12 in]
        "RH :" <- w4546
        n3489 = Equal?(x=w4546, y=0.0) -> (x = y?=w4549:bool)
        n3490 = case shown="False" w4549 {
          tunnel: [w4566 w4567] -> w4550
          tunnel: w4546 -> [w4566 _]
          frame False {
            "Humidity temp 2" <- w4566
          }
          frame True {
            n3491 = local read "Humidity temp 2"() -> (w4567:dbl)
          }
        }
        n3492 = local write "RH Numeric:"(w4550) -> ()
      }
    }
    n3493 = local read "Quit"() -> (w4516:bool)
  }
  n3494 = while {
    shift-right: [w4573] -> _
    shift-left: _ -> [w4574]
    shift-right: [w4571] -> _
    shift-left: T20 {"Read Uno"="", "Bytes at Heave Port"=0.0, "UNO COM Port:"="COM9", "UNO COM Port: 2"="COM7", "Residual Due"="", "UNO COM Status 2"=TRUE, "UNO COM Status"=TRUE, "Port 2"=TRUE, "Sway PPR"=6400.0, "Surge PPR"=6400.0, "Heave PPR"=6400.0, "Sway Pitch"=2.0, "Surge Pitch"=3.0, "Heave Pitch"=4.0, "Sway Pulses/mm"=320.0, "Surge Pulses/mm"=1600.0, "Heave Pulses/mm"=1600.0, "inner loop"=0.0, "Read Heave and Surge 2"="", "String 36"="", "Write S"=FALSE, "WriteCC1"=[""], "Heave COM Loop"=0, "LastCom"="", "EXIT"=FALSE, "Error Heave"={"status"=TRUE, "code"=-1073807343, "source"=""}} -> [w4570]
    shift-right: [w4568] -> _
    shift-left: enum16{"init", "MAIN", "Panel Close"}."init" -> [w4569]
    stop <- w4572 stop-if-true
    # "UNO CODE LOGIC"
    n3495 = case shown="\"MAIN\"" w4569 {
      tunnel: w4574 -> [w4588 w4607 w4663 w4665]
      tunnel: [w4583 w4612 w4663 w4665] -> w4573
      tunnel: [_ _ TRUE _] -> w4572
      tunnel: [w4579 w4610 w4661 w4664] -> w4571
      tunnel: w4570 -> [w4585 w4606 w4661 w4664]
      tunnel: [enum16{"init", "MAIN", "Panel Close"}."MAIN" w4601 _ _] -> w4568
      frame "init" {
        n3496 = local read "Com Port 1"() -> (w4575:refnum<visa-resource-name>)
        n3497 = Bundle By Name(cluster=w4585, "UNO COM Port:"=w4575) -> (w4584:T20)
        n3498 = call "Instrument fgv.vi"("Enum"=T32."INIT", "error in (no error) 2"=w4588, "INPUT"=w4584) -> ("error"=w4586:errorcluster, "output"=w4582:T18)  [unwired: 6 in, 1 out]
        n3499 = case shown="Error" w4586 {
          selector: w4586 -> [w4590 _]
          tunnel: [w4590 w4594] -> w4583
          tunnel: w4582 -> [w4589 w4592]
          tunnel: [w4589 w4591] -> w4580
          frame No Error {
          }
          frame Error {
            n3500 = call "Instrument fgv.vi"("Enum"=T32."ERROR INIT", "INPUT"=w4592) -> ("error"=w4595:errorcluster, "output"=w4591:T18)  [unwired: 7 in, 1 out]
            n3501 = call <vilib>:"Clear Errors.vi"("error in (no error)"=w4595) -> ("error out"=w4594:errorcluster)  [unwired: 5 in, 1 out]
          }
        }
        n3502 = local read "LastCom UNO"() -> (w4577:string)
        n3503 = Unbundle By Name(w4580) -> ("Heave COM Status 2"=→"Instrument Status":bool, "Error Heave"=→"Error  2":errorcluster)  [unwired: 1 out]
        n3504 = Bundle By Name(cluster=w4580, "LastCom"=w4577) -> (w4579:T18)
      }
      frame "MAIN" {
        n3505 = Unbundle By Name(w4606) -> ("UNO COM Port: 2"=w4596:refnum<visa-resource-name>)
        n3506 = local read "Com Port 1"() -> (w4597:refnum<visa-resource-name>)
        n3507 = local write "COM Port UNO :"(w4596) -> ()
        n3508 = Equal?(x=w4596, y=w4597) -> (x = y?=w4613:bool)
        n3509 = Bundle By Name(cluster=w4606, "UNO COM Port:"=w4597) -> (w4605:T20)
        n3510 = case shown="True" w4613 {
          tunnel: [w4617 w4634] -> w4612
          tunnel: w4607 -> [w4618 w4640]
          tunnel: w4605 -> [w4616 w4638]
          tunnel: [w4615 w4633] -> w4610
          frame False {
            n3511 = call <vilib>:"Clear Errors.vi"("error in (no error)"=w4618) -> ("error out"=w4614:errorcluster)  [unwired: 5 in, 1 out]
            n3512 = call "Instrument fgv.vi"("Enum"=T32."ERROR INIT", "error in (no error) 2"=w4614, "INPUT"=w4616) -> ("error"=w4620:errorcluster, "output"=w4615:T18)  [unwired: 6 in, 1 out]
            n3513 = call <vilib>:"Clear Errors.vi"("error in (no error)"=w4620) -> ("error out"=w4617:errorcluster)  [unwired: 5 in, 1 out]
          }
          frame True {
            n3514 = call "Instrument fgv.vi"("Enum"=T32."READ", "error in (no error) 2"=w4640, "INPUT"=w4638) -> ("error"=w4639:errorcluster, "output"=w4632:T18)  [unwired: 6 in, 1 out]
            n3515 = Bundle By Name(cluster=w4632, "String 36"="WRITE UNO") -> (w4631:T18)
            n3516 = case shown="True" "Write" {
              selector: "Write" -> [_ w4655]
              tunnel: w4639 -> [w4653 w4660]
              tunnel: [w4653 w4659] -> w4629
              tunnel: w4631 -> [w4652 w4657]
              tunnel: [w4652 w4656] -> w4628
              frame False {
              }
              frame True {
                n3517 = Not(x=w4655) -> (.not. x?=w4654:bool)
                n3518 = local write "Write"(w4654) -> ()
                n3519 = call "Instrument fgv.vi"("Enum"=T32."MANUAL WRITE", "error in (no error) 2"=w4660, "INPUT"=w4657) -> ("error"=w4659:errorcluster, "output"=w4656:T18)  [unwired: 6 in, 1 out]
              }
            }
            n3520 = Array Size(array="Write UNO") -> (size(s)=w4626:i32)
            n3521 = Greater Than 0?(x=w4626) -> (x > 0?=w4625:bool)
            n3522 = call "Instrument fgv.vi"("Enum"=T32."WRITE", "error in (no error) 2"=w4629, "WriteCC1"="Write UNO", "INPUT"=w4628) -> ("error"=w4636:errorcluster, "WriteCC1 2"=w4627:string[], "output"=w4635:T18)  [unwired: 5 in]
            n3523 = case shown="True" w4625 {
              tunnel: w4627 -> [_ w4642]
              frame False {
              }
              frame True {
                n3524 = local write "Write UNO"(w4642) -> ()
              }
            }
            n3525 = case shown="Error" w4636 {
              selector: w4636 -> [w4643 w4646]
              tunnel: w4635 -> [w4644 w4651]
              tunnel: [w4644 w4650] -> w4633
              tunnel: [w4643 w4648] -> w4634
              frame No Error {
              }
              frame Error {
                n3526 = call <vilib>:"Clear Errors.vi"("error in (no error)"=w4646) -> ("error out"=w4645:errorcluster)  [unwired: 5 in, 1 out]
                n3527 = call "Instrument fgv.vi"("Enum"=T32."ERROR INIT", "error in (no error) 2"=w4645, "INPUT"=w4651) -> ("error"=w4649:errorcluster, "output"=w4650:T18)  [unwired: 6 in, 1 out]
                n3528 = call <vilib>:"Clear Errors.vi"("error in (no error)"=w4649) -> ("error out"=w4648:errorcluster)  [unwired: 5 in, 1 out]
              }
            }
            n3529 = Unbundle By Name(w4633) -> ("LastCom"=→"LastCom UNO":string, "Read Heave and Surge"=→"Read UNO":string)
          }
        }
        n3530 = Unbundle By Name(w4610) -> ("Heave COM Status 2"=w4611:bool, "Heave COM Status"=w4600:bool, "Error Heave"=w4598:errorcluster, "Bytes at Heave Port"=→"Bytes at Humidity Port":dbl)
        n3531 = Not(x=w4600) -> (.not. x?=w4608:bool)
        n3532 = Not(x=w4611) -> (.not. x?=w4599:bool)
        n3533 = local write "Instrument Status"(w4608) -> ()
        n3534 = local write "Error  2"(w4598) -> ()
        n3535 = local write "Port 1a"(w4600) -> ()
        n3536 = local read "Quit"() -> (w4602:bool)
        n3537 = local write "COM Status"(w4599) -> ()
        n3538 = Select(t=enum16{"init", "MAIN", "Panel Close"}."Panel Close", s=w4602, f=enum16{"init", "MAIN", "Panel Close"}."MAIN") -> (s? t:f=w4601:enum16{"init", "MAIN", "Panel Close"})
      }
      frame "Panel Close" {
      }
      frame Default {
      }
    }
  }
